vi "TLB Native Dynamic Events ver 0.26e.vi"() -> ()   [LabVIEW 2018] (continued)
      tunnel: [w3002 w3015 w3027 w3042 w3061 w3076 w3091 w3105 w3119 w3135 w3150 w3164 w3175 w3192 w3210 w3228 w3251 w3263 w3276 w3305 w3318 w3331 w3346 w3357 w3373 w3393 w3428 w3462 w3475 w3488 w3499 w3511 w3527 w3543 w3555 w3568 w3602 w3613 w3625 w3657 w3668 w3679 w3692 w3705 w3718 w3731 w3744 w3759 w3775 w3788 w3804 w3820 w3836 w3853 w3866 w3886 w3906] -> w237
      tunnel: [_ _ _ _ _ _ _ _ _ _ _ _ _ _ _ _ _ _ _ _ _ _ _ _ _ _ _ _ _ _ _ _ _ _ _ w3567 w3597 _ _ _ _ _ _ _ _ _ _ _ _ _ _ _ _ _ _ _ _] -> w235
      tunnel: w233 -> [w3001 w3014 w3026 w3041 w3060 w3075 w3090 w3104 w3118 w3134 w3149 w3163 w3174 w3191 w3209 w3227 w3243 w3262 w3274 w3304 w3317 w3330 w3345 w3356 w3375 w3395 w3430 w3461 w3474 w3487 w3498 w3510 w3526 w3542 w3554 w3566 w3601 w3612 w3624 w3656 w3667 w3678 w3691 w3704 w3717 w3730 w3743 w3758 w3774 w3787 w3803 w3819 w3835 w3852 w3865 w3885 w3905]
      tunnel: [w3001 w3014 w3026 w3041 w3060 w3075 w3090 w3104 w3118 w3134 w3149 w3163 w3174 w3191 w3209 w3227 w3243 w3262 w3274 w3304 w3317 w3330 w3345 w3356 w3375 w3395 w3430 w3461 w3474 w3487 w3498 w3510 w3526 w3542 w3554 w3566 w3601 w3612 w3624 w3656 w3667 w3678 w3691 w3704 w3717 w3730 w3743 w3758 w3774 w3787 w3803 w3819 w3835 w3852 w3865 w3885 w3905] -> w232
      tunnel: w228 -> [w3000 w3013 w3025 w3040 w3059 w3074 w3089 w3103 w3117 w3133 w3148 w3162 w3173 w3190 w3208 w3224 w3242 w3261 w3273 w3303 w3316 w3329 w3344 w3355 w3370 w3388 w3423 w3460 w3473 w3486 w3497 w3509 w3525 w3541 w3553 w3565 w3595 w3611 w3623 w3655 w3666 w3677 w3690 w3703 w3716 w3729 w3742 w3757 w3773 w3786 w3802 w3818 w3834 w3851 w3864 w3884 w3899]
      tunnel: [w3000 w3013 w3025 w3040 w3059 w3074 w3089 w3103 w3117 w3133 w3148 w3162 w3173 w3190 w3208 w3224 w3242 w3261 w3273 w3303 w3316 w3329 w3344 w3355 w3369 w3388 w3423 w3460 w3473 w3486 w3497 w3509 w3525 w3541 w3553 w3565 w3588 w3611 w3623 w3654 w3666 w3677 w3690 w3703 w3716 w3729 w3742 w3757 w3773 w3786 w3802 w3818 w3834 w3851 w3864 w3884 w3898] -> w227
      frame "Exit" {
        # ">>State Logic  >>"
        # ">>> Time cluster >>>"
        # ">>> Yaw >>>"
        # ">>> Stepper position >>>"
        # ">>> Encoders >>>"
        # ">>> Object detection >>>"
        # ">>> Ultrasonic Sensors Detect >>>"
        n75 = call "Imaq Dispose"("All Images? (No)"=TRUE) -> ()  [unwired: 5 in, 1 out]
      }
      frame "----Movement States----" {
        # ">>State Logic  >>"
        # ">>> Time cluster >>>"
        # ">>> Yaw >>>"
        # ">>> Stepper position >>>"
        # ">>> Encoders >>>"
        # ">>> Object detection >>>"
        # ">>> Ultrasonic Sensors Detect >>>"
      }
      frame "FORWARD" {
        # ">>State Logic  >>"
        # ">>> Time cluster >>>"
        # ">>> Yaw >>>"
        # ">>> Stepper position >>>"
        # ">>> Encoders >>>"
        # ">>> Object detection >>>"
        # ">>> Ultrasonic Sensors Detect >>>"
        n76 = Unbundle By Name(w3033) -> ("Yaw"=w3029:dbl)
        n77 = call "MOTOR CONTROL WITH PID AE.vi"("Yaw"=w3029, "Speed"=40.0, "Direction"=MOTOR_CONTROL_WITH_PID_AE_DIRECTION_TYPE_DEF."y-axis movement", "AE Mode"=MOTOR_CONTROL_WITH_PID_AE_DATA_MODE_TYPE_DEF."Write to AE") -> ()  [unwired: 1 out]
      }
      frame "FORWARD - IR ASSIST" {
        # "Algorithm sensitivity"
        # "Distance to maintain from wall"
        # ">>State Logic  >>"
        # ">>> Time cluster >>>"
        # ">>> Yaw >>>"
        # ">>> Stepper position >>>"
        # ">>> Encoders >>>"
        # ">>> Object detection >>>"
        # ">>> Ultrasonic Sensors Detect >>>"
        n78 = Unbundle By Name(w3048) -> ("Left IR Sensor"=w3047:dbl)
        n79 = Subtract(x=w3047, y=10.0) -> (x-y=w3045:dbl)
        n80 = Multiply(x=w3045, y=0.2) -> (x*y=w3043:dbl)
        n81 = call "MOTOR CONTROL WITH PID AE.vi"("Yaw"=w3043, "Speed"=35.0, "Direction"=MOTOR_CONTROL_WITH_PID_AE_DIRECTION_TYPE_DEF."y-axis movement", "AE Mode"=MOTOR_CONTROL_WITH_PID_AE_DATA_MODE_TYPE_DEF."Write to AE") -> ()  [unwired: 1 out]
      }
      frame "LEFT" {
        # ">>State Logic  >>"
        # ">>> Time cluster >>>"
        # ">>> Yaw >>>"
        # ">>> Stepper position >>>"
        # ">>> Encoders >>>"
        # ">>> Object detection >>>"
        # ">>> Ultrasonic Sensors Detect >>>"
        n82 = Unbundle By Name(w3067) -> ("Yaw"=w3064:dbl)
        n83 = call "MOTOR CONTROL WITH PID AE.vi"("Yaw"=w3064, "Speed"=-20.0, "Direction"=MOTOR_CONTROL_WITH_PID_AE_DIRECTION_TYPE_DEF."x-axis movement", "AE Mode"=MOTOR_CONTROL_WITH_PID_AE_DATA_MODE_TYPE_DEF."Write to AE") -> ()  [unwired: 1 out]
      }
      frame "RIGHT" {
        # ">>> Time cluster >>>"
        # ">>> Yaw >>>"
        # ">>> Stepper position >>>"
        # ">>> Encoders >>>"
        # ">>> Object detection >>>"
        # ">>> Ultrasonic Sensors Detect >>>"
        n84 = Unbundle By Name(w3082) -> ("Yaw"=w3078:dbl)
        n85 = call "MOTOR CONTROL WITH PID AE.vi"("Yaw"=w3078, "Speed"=30.0, "Direction"=MOTOR_CONTROL_WITH_PID_AE_DIRECTION_TYPE_DEF."x-axis movement", "AE Mode"=MOTOR_CONTROL_WITH_PID_AE_DATA_MODE_TYPE_DEF."Write to AE") -> ()  [unwired: 1 out]
      }
      frame "R-ACW" {
        # ">>> IR Sensors >>>"
        # ">>> Time cluster >>>"
        # ">>> Yaw >>>"
        # ">>> Stepper position >>>"
        # ">>> Encoders >>>"
        # ">>> Object detection >>>"
        # ">>> Ultrasonic Sensors Detect >>>"
        n86 = call "MOTOR CONTROL WITH PID AE.vi"("Speed"=10.0, "Direction"=MOTOR_CONTROL_WITH_PID_AE_DIRECTION_TYPE_DEF."rotation", "AE Mode"=MOTOR_CONTROL_WITH_PID_AE_DATA_MODE_TYPE_DEF."Write to AE") -> ()  [unwired: 1 in, 1 out]
      }
      frame "R-CW" {
        (unwired) -0.2 ("Speed")
        # ">>> Time cluster >>>"
        # ">>> Yaw >>>"
        # ">>> Stepper position >>>"
        # ">>> Encoders >>>"
        # ">>> Object detection >>>"
        # ">>> Ultrasonic Sensors Detect >>>"
        n87 = call "MOTOR CONTROL WITH PID AE.vi"("Speed"=-10.0, "Direction"=MOTOR_CONTROL_WITH_PID_AE_DIRECTION_TYPE_DEF."rotation", "AE Mode"=MOTOR_CONTROL_WITH_PID_AE_DATA_MODE_TYPE_DEF."Write to AE") -> ()  [unwired: 1 in, 1 out]
      }
      frame "X AXIS - SLOW" {
        # ">>> Line Sensor Cluster>>>"
        # ">>> IR Sensors >>>"
        # ">>> Time cluster >>>"
        # ">>> Yaw >>>"
        # ">>> Stepper position >>>"
        # ">>> Encoders >>>"
        # ">>> Object detection >>>"
        # ">>> Ultrasonic Sensors Detect >>>"
        n88 = Unbundle By Name(w3121) -> ("xSpeed"=w3120:dbl)
        n89 = Unbundle By Name(w3126) -> ("Yaw"=w3123:dbl)
        n90 = call "MOTOR CONTROL WITH PID AE.vi"("Yaw"=w3123, "Speed"=w3120, "Direction"=MOTOR_CONTROL_WITH_PID_AE_DIRECTION_TYPE_DEF."x-axis movement", "AE Mode"=MOTOR_CONTROL_WITH_PID_AE_DATA_MODE_TYPE_DEF."Write to AE") -> ()  [unwired: 1 out]
      }
      frame "REVERSE" {
        # ">>> Time cluster >>>"
        # ">>> Yaw >>>"
        # ">>> Stepper position >>>"
        # ">>> Encoders >>>"
        # ">>> Object detection >>>"
        # ">>> Ultrasonic Sensors Detect >>>"
        n91 = Unbundle By Name(w3141) -> ("Yaw"=w3137:dbl)
        n92 = call "MOTOR CONTROL WITH PID AE.vi"("Yaw"=w3137, "Speed"=-50.0, "Direction"=MOTOR_CONTROL_WITH_PID_AE_DIRECTION_TYPE_DEF."y-axis movement", "AE Mode"=MOTOR_CONTROL_WITH_PID_AE_DATA_MODE_TYPE_DEF."Write to AE") -> ()  [unwired: 1 out]
      }
      frame "STOP" {
        n93 = Wait (ms)(milliseconds to wait=u32 100) -> ()  [unwired: 1 out]
        n94 = call "MOTOR CONTROL WITH PID AE.vi"("Direction"=MOTOR_CONTROL_WITH_PID_AE_DIRECTION_TYPE_DEF."stop", "AE Mode"=MOTOR_CONTROL_WITH_PID_AE_DATA_MODE_TYPE_DEF."Write to AE") -> ()  [unwired: 2 in, 1 out]
      }
      frame "----SENSOR READING---- " {
      }
      frame "READ ENCODERS" {
        # ">>> Time cluster >>>"
        # ">>> Yaw >>>"
        # ">>> Stepper position >>>"
        # ">>> Object detection >>>"
        # ">>> Current encoder distance >>>"
        # ">>> Ultrasonic Sensors Detect >>>"
        n95 = call "MOTOR CONTROL WITH PID AE.vi"("AE Mode"=MOTOR_CONTROL_WITH_PID_AE_DATA_MODE_TYPE_DEF."Read from AE") -> ("Speed & distance"=w3180:T15)  [unwired: 3 in]
        n96 = Unbundle By Name(w3180) -> ("xDistance"=w3179:dbl, "yDistance"=w3178:dbl, "wDistance"=w3177:dbl)
        n97 = Bundle By Name(cluster=w3187, "xDistance"=w3179, "yDistance"=w3178, "wDistance"=w3177) -> (w3186:T8)
      }
      frame "READ ULTRASONIC" {
        (unwired) navX_type_def."Read Values" ("Mode")
        (unwired) MOTOR_CONTROL_NO_PID_Type_Def."Latch" ("Direction")
        # ">>> Line Sensor Cluster>>>"
        # ">>> IR Sensors >>>"
        # ">>State Logic  >>"
        # ">>> Time cluster >>>"
        # ">>> Ultrasonic Sensors Detect >>>"
        # ">>> Object detection >>>"
        # ">>> Encoders >>>"
        # ">>> Stepper position >>>"
        # ">>> Yaw >>>"
        n98 = call "Arduino Interfacing VI.vi"("AE Mode"=Arduino_Interfacing."Read From Arduino") -> ("Arduino Data"=w3200:T17)  [unwired: 3 in, 1 out]
        n99 = Unbundle By Name(w3200) -> ("PING A"=w3199:u8, "PING B"=w3198:u8, "PING C"=w3197:u8, "PING D"=w3196:u8)
        n100 = Bundle By Name(cluster=w3206, "PING_A"=w3199, "PING_B"=w3198, "PING_C"=w3197, "PING_D"=w3196) -> (w3207:T9)
      }
      frame "READ NAVX" {
        # ">> Item Selection Bias >>"
        # ">>State Logic  >>"
        # ">>> Line Sensor Cluster>>>"
        # ">>> IR Sensors >>>"
        # ">>> Time cluster >>>"
        # ">>> Yaw >>>"
        # ">>> Ultrasonic Sensors Detect >>>"
        # ">>> Object detection >>>"
        # ">>> Encoders >>>"
        # ">>> Stepper position >>>"
        n101 = call "navX reading VI.vi"("Mode"=navX_type_def."Read Values") -> ("NavX Readings"=w3213:T16)  [unwired: 2 in, 3 out]
        n102 = Unbundle By Name(w3213) -> ("Heading"=w3212:dbl)
        n103 = Unbundle By Name(w3213) -> ("Yaw"=w3216:dbl)
        n104 = Bundle By Name(cluster=w3218, "Yaw"=w3216, "Compass"=w3212) -> (w3217:T6)
      }
      frame "READ IR" {
        w3226 = T41 [enum."B/AI2"] items=["Not Connected", "AudioIn/Left", "AudioIn/Right", "C/AI0", "C/AI1", "A/AI0", "A/AI1", "A/AI2", "A/AI3", "A/AI4", "A/AI5", "A/AI6", "A/AI7", "B/AI0", "B/AI1", "B/AI2", "B/AI3", "B/AI4", "B/AI5", "B/AI6", "B/AI7", "AI/AI0", "AI/AI1", "AI/AI2", "AI/AI3", "A/AI0 (DIFF)", "A/AI1 (DIFF)", "A/AI2 (DIFF)", "A/AI3 (DIFF)", "B/AI0 (DIFF)", "B/AI1 (DIFF)", "B/AI2 (DIFF)", "B/AI3 (DIFF)"] ("AI Channel")
        w3230 = T41 [enum."B/AI1"] items=["Not Connected", "AudioIn/Left", "AudioIn/Right", "C/AI0", "C/AI1", "A/AI0", "A/AI1", "A/AI2", "A/AI3", "A/AI4", "A/AI5", "A/AI6", "A/AI7", "B/AI0", "B/AI1", "B/AI2", "B/AI3", "B/AI4", "B/AI5", "B/AI6", "B/AI7", "AI/AI0", "AI/AI1", "AI/AI2", "AI/AI3", "A/AI0 (DIFF)", "A/AI1 (DIFF)", "A/AI2 (DIFF)", "A/AI3 (DIFF)", "B/AI0 (DIFF)", "B/AI1 (DIFF)", "B/AI2 (DIFF)", "B/AI3 (DIFF)"] ("AI Channel")
        w3235 = T41 [enum."B/AI0"] items=["Not Connected", "AudioIn/Left", "AudioIn/Right", "C/AI0", "C/AI1", "A/AI0", "A/AI1", "A/AI2", "A/AI3", "A/AI4", "A/AI5", "A/AI6", "A/AI7", "B/AI0", "B/AI1", "B/AI2", "B/AI3", "B/AI4", "B/AI5", "B/AI6", "B/AI7", "AI/AI0", "AI/AI1", "AI/AI2", "AI/AI3", "A/AI0 (DIFF)", "A/AI1 (DIFF)", "A/AI2 (DIFF)", "A/AI3 (DIFF)", "B/AI0 (DIFF)", "B/AI1 (DIFF)", "B/AI2 (DIFF)", "B/AI3 (DIFF)"] ("AI Channel")
        # ">>> Line Sensor Cluster>>>"
        # ">>> IR Sensors >>>"
        # ">>State Logic  >>"
        # ">>> Time cluster >>>"
        # ">>> Ultrasonic Sensors Detect >>>"
        # ">>> Object detection >>>"
        # ">>> Encoders >>>"
        # ">>> Stepper position >>>"
        # ">>> Yaw >>>"
        n105 = call <vilib>:"Sharp IR.vi"("AI Channel"=w3235) -> ("Sharp IR Distance"=w3231:dbl)  [unwired: 8 in, 2 out]
        n106 = call <vilib>:"Sharp IR.vi"("AI Channel"=w3230) -> ("Sharp IR Distance"=w3229:dbl)  [unwired: 8 in, 2 out]
        n107 = call <vilib>:"Sharp IR.vi"("AI Channel"=w3226) -> ("Sharp IR Distance"=w3225:dbl)  [unwired: 8 in, 2 out]
        n108 = Bundle By Name(cluster=w3233, "Left IR Sensor"=w3231, "Arm IR Sensor"=w3229, "Bottom IR Sensor"=w3225) -> (w3232:T5)
      }
      frame "READ LINE SENSOR" {
        # ">>> IR Sensors >>>"
        # ">>> Line Sensor Cluster>>>"
        # ">>State Logic  >>"
        # ">>> Time cluster >>>"
        # ">>> Object detection >>>"
        # ">>> Yaw >>>"
        # ">>> Ultrasonic Sensors Detect >>>"
        # ">>> Encoders >>>"
        # ">>> Stepper position >>>"
        n109 = call "Line Sensor AE.vi"("AE State"=Line_Sensor_AE_Type_Def."READ FROM LINE SENSORS") -> ("Line Detected?"=w3249:bool, "Line Sensor Raw Values"=w3248:T43)
        n110 = Unbundle By Name(w3248) -> ("S1"=w3247:dbl, "S2"=w3246:dbl, "S3"=w3245:dbl, "S4"=w3244:dbl)
        n111 = Bundle By Name(cluster=w3252, "Line Detected?"=w3249, "S1"=w3247, "S2"=w3246, "S3"=w3245, "S4"=w3244) -> (w3251:T4)
      }
      frame "----SYSTEM MODES----" {
        (unwired) I2C_MASTER_Type_Def."Last State" ("Arduino Mode")
        # ">>> Object detection >>>"
        # ">>> Yaw >>>"
        # ">>> Ultrasonic Sensors Detect >>>"
        # ">>> Encoders >>>"
        # ">>> Stepper position >>>"
      }
      frame "INIT" {
        w3296 = u8 0
        w3297 = 0.0
        # ">>> IR Sensors >>>"
        # ">>> IR Sensors >>>"
        # ">>> Line Sensor Cluster>>>"
        # ">>> Time cluster >>>"
        # ">>> Object detection >>>"
        # ">>> Yaw >>>"
        # ">>> Ultrasonic Sensors Detect >>>"
        # ">>> Encoders >>>"
        # ">>> Stepper position >>>"
        # ">>State Logic  >>"
        n112 = call "Arduino Interfacing VI.vi"("AE Mode"=Arduino_Interfacing."Initialize") -> ()  [unwired: 3 in, 2 out]
        n113 = call "FGV Stop.vi"("Init/Read/Write State"=States_for_Action_Engine."Initialize") -> ()  [unwired: 2 in, 2 out]
        n114 = call "Elasped Timer.vi"("Action"=Elapsed_timer_control."Initialize") -> ()  [unwired: 7 in, 4 out]
        n115 = call "MOTOR CONTROL WITH PID AE.vi"("AE Mode"=MOTOR_CONTROL_WITH_PID_AE_DATA_MODE_TYPE_DEF."Init AE") -> ()  [unwired: 3 in, 1 out]
        n116 = call "IMAQ Reference AE.vi"("IMAQ AE States"=IMAQ_Reference_AE."Initialize AE") -> ()  [unwired: 1 in, 2 out]
        n117 = call "Line Sensor AE.vi"("AE State"=Line_Sensor_AE_Type_Def."INIT AE") -> ()  [unwired: 2 out]
        n118 = Bundle By Name(cluster=w3290, "Recognized Object"=FALSE, "Object X coordinate"=0.0, "Object Y coordinate"=0.0) -> (w3289:T11)
        n119 = Bundle By Name(cluster=w3295, "y Stepper Position"=u8 0, "z Stepper Position"=u8 0) -> (w3294:T7)
        n120 = Bundle By Name(cluster=w3299, "xDistance"=w3297, "yDistance"=w3297, "wDistance"=w3297) -> (w3298:T8)
        n121 = Bundle By Name(cluster=w3301, "PING_A"=w3296, "PING_B"=w3296, "PING_C"=w3296, "PING_D"=w3296) -> (w3302:T9)
        n122 = invoke class="VI" method="Default Vals.Reinit All"() -> ()  [unwired: 3 in, 3 out]
        n123 = Bundle By Name(cluster=w3285, "Yaw"=0.0) -> (w3284:T6)
        n124 = call "Box Colour FGV.vi"("Init/R/W State"=Box_Colour_FGV_States."Initialize") -> ()  [unwired: 9 in, 2 out]
      }
      frame "ARDUINO - ULTRASONIC" {
        # ">>> Time cluster >>>"
        # ">>> Line Sensor Cluster>>>"
        # ">>> Object detection >>>"
        # ">>> Yaw >>>"
        # ">>> Ultrasonic Sensors Detect >>>"
        # ">>> Encoders >>>"
        # ">>> Stepper position >>>"
        # ">>State Logic  >>"
        n125 = call "Arduino Interfacing VI.vi"("Data to Write"=I2C_MASTER_WRITE_NEW_Type_Def."Ultrasonic sensors", "AE Mode"=Arduino_Interfacing."Write to Arduino") -> ()  [unwired: 2 in, 2 out]
      }
      frame "NAVX CALIBRATE" {
        # ">>> Object detection >>>"
        # ">>> Yaw >>>"
        # ">>> Ultrasonic Sensors Detect >>>"
        # ">>> Encoders >>>"
        # ">>> Stepper position >>>"
        # ">>State Logic  >>"
        # "Adds a 15 second delay to the startup process \nfor the NavX to calibrate"
        n126 = Wait (ms)(milliseconds to wait=u32 1000) -> ()  [unwired: 1 out]
      }
      frame "NO ACTION", Default {
        (unwired) u8 0 ("y Stepper value")
        (unwired) TRUE ("Latch")
        (unwired) navX_type_def."Read Values" ("Mode")
        (unwired) MOTOR_CONTROL_NO_PID_Type_Def."Latch" ("Direction")
        # ">>> Object detection >>>"
        # ">>> Yaw >>>"
        # ">>> Ultrasonic Sensors Detect >>>"
        # ">>> Encoders >>>"
        # ">>> Stepper position >>>"
        # ">>State Logic  >>"
        n127 = case shown="4" w3338 {
          tunnel: [0 100] -> w3340
          frame 1, Default {
          }
          frame 4 {
          }
        }
      }
      frame "----RESET CASES----" {
        (unwired) I2C_MASTER_Type_Def."Last State" ("Arduino Mode")
        # ">>> Object detection >>>"
        # ">>> Yaw >>>"
        # ">>> Ultrasonic Sensors Detect >>>"
        # ">>> Encoders >>>"
        # ">>> Stepper position >>>"
        # ">>State Logic  >>"
      }
      frame "RESET ENCODERS" {
        # ">>> Object detection >>>"
        # ">>> Yaw >>>"
        # ">>> Ultrasonic Sensors Detect >>>"
        # ">>> Encoders >>>"
        # ">>> Stepper position >>>"
        # ">>State Logic  >>"
        n128 = call "MOTOR CONTROL WITH PID AE.vi"("Direction"=MOTOR_CONTROL_WITH_PID_AE_DIRECTION_TYPE_DEF."reset encoders", "AE Mode"=MOTOR_CONTROL_WITH_PID_AE_DATA_MODE_TYPE_DEF."Write to AE") -> ()  [unwired: 2 in, 1 out]
      }
      frame "RESET FLAGS" {
        w3368 = FALSE ("Line Detected?")
        # ">>> Line Sensor Cluster>>>"
        # ">>> IR Sensors >>>"
        # ">>> Time cluster >>>"
        # ">>> Object detection >>>"
        # ">>> Yaw >>>"
        # ">>> Ultrasonic Sensors Detect >>>"
        # ">>> Encoders >>>"
        # ">>> Stepper position >>>"
        # ">>> Line Sensor Cluster>>>"
        # ">>> IR Sensors >>>"
        # ">>> Time cluster >>>"
        # ">>> Object detection >>>"
        # ">>> Yaw >>>"
        # ">>> Ultrasonic Sensors Detect >>>"
        # ">>> Encoders >>>"
        # ">>> Stepper position >>>"
        # "Resets BOOLEAN FLAGS only"
        n129 = Wait (ms)(milliseconds to wait=u32 20) -> ()  [unwired: 1 out]
        n130 = Bundle By Name(cluster=w3384, "Recognized Object"=FALSE) -> (w3383:T11)
        n131 = Bundle By Name(cluster=w3374, "Line Detected?"=FALSE) -> (w3373:T4)
        n132 = Bundle By Name(cluster=w3378, "Time up flag"=FALSE) -> (w3377:T3)
        n133 = Bundle By Name(cluster=w3370, "Red"=w3368, "Black"=w3368, "Blue"=w3368, "Yellow"=w3368, "Green"=w3368, "Unknown"=w3368, "Image processing done"=w3368) -> (w3369:T1)
      }
      frame "RESET SENSOR VALUES" {
        w3389 = 0.0 ("S4")
        w3390 = 0.0 ("S4")
        # "Resets SENSOR VALUES only"
        # ">>> Line Sensor Cluster>>>"
        # ">>> IR Sensors >>>"
        # ">>> Time cluster >>>"
        # ">>> Object detection >>>"
        # ">>> Yaw >>>"
        # ">>> Ultrasonic Sensors Detect >>>"
        # ">>> Encoders >>>"
        # ">>> Stepper position >>>"
        # ">>> Line Sensor Cluster>>>"
        # ">>> IR Sensors >>>"
        # ">>> Time cluster >>>"
        # ">>> Object detection >>>"
        # ">>> Yaw >>>"
        # ">>> Ultrasonic Sensors Detect >>>"
        # ">>> Encoders >>>"
        # ">>> Stepper position >>>"
        # "Resets any software variables\nand/or non-critical states"
        n134 = Wait (ms)(milliseconds to wait=u32 20) -> ()  [unwired: 1 out]
        n135 = Bundle By Name(cluster=w3398, "SET TIME TO CHECK"=0.0) -> (w3397:T3)
        n136 = Bundle By Name(cluster=w3414, "Object X coordinate"=0.0, "Object Y coordinate"=0.0) -> (w3413:T11)
        n137 = Bundle By Name(cluster=w3405, "y Stepper Position"=u8 0, "z Stepper Position"=u8 0) -> (w3404:T7)
        n138 = Bundle By Name(cluster=w3392, "Left IR Sensor"=w3389, "Arm IR Sensor"=w3389) -> (w3391:T5)
        n139 = Bundle By Name(cluster=w3410, "xDistance"=0.0, "yDistance"=0.0, "wDistance"=0.0) -> (w3409:T8)
        n140 = Bundle By Name(cluster=w3421, "PING_A"=u8 0, "PING_B"=u8 0, "PING_C"=u8 0, "PING_D"=u8 0) -> (w3420:T9)
        n141 = Bundle By Name(cluster=w3401, "Yaw"=0.0) -> (w3400:T6)
        n142 = Bundle By Name(cluster=w3394, "S1"=w3390, "S2"=w3390, "S3"=w3390, "S4"=w3390) -> (w3393:T4)
      }
      frame "RESET ALL SENSORS" {
        w3424 = 0.0 ("SET TIME TO CHECK")
        # ">>> Line Sensor Cluster>>>"
        # ">>> IR Sensors >>>"
        # ">>> Time cluster >>>"
        # ">>> Object detection >>>"
        # ">>> Yaw >>>"
        # ">>> Ultrasonic Sensors Detect >>>"
        # ">>> Encoders >>>"
        # ">>> Stepper position >>>"
        # ">>> Line Sensor Cluster>>>"
        # ">>> IR Sensors >>>"
        # ">>> Time cluster >>>"
        # ">>> Object detection >>>"
        # ">>> Yaw >>>"
        # ">>> Ultrasonic Sensors Detect >>>"
        # ">>> Encoders >>>"
        # ">>> Stepper position >>>"
        # "Resets ALL SENSOR PARAMTERS"
        n143 = Wait (ms)(milliseconds to wait=u32 20) -> ()  [unwired: 1 out]
        n144 = Bundle By Name(cluster=w3434, "Time up flag"=FALSE, "SET TIME TO CHECK"=0.0) -> (w3433:T3)
        n145 = Bundle By Name(cluster=w3451, "Recognized Object"=FALSE, "Object X coordinate"=0.0, "Object Y coordinate"=0.0) -> (w3450:T11)
        n146 = Bundle By Name(cluster=w3441, "y Stepper Position"=u8 0, "z Stepper Position"=u8 0) -> (w3440:T7)
        n147 = Bundle By Name(cluster=w3429, "Line Detected?"=FALSE) -> (w3428:T4)
        n148 = Bundle By Name(cluster=w3426, "Left IR Sensor"=w3424, "Arm IR Sensor"=w3424) -> (w3425:T5)
        n149 = Bundle By Name(cluster=w3446, "xDistance"=0.0, "yDistance"=0.0, "wDistance"=0.0) -> (w3445:T8)
        n150 = Bundle By Name(cluster=w3458, "PING_A"=u8 0, "PING_B"=u8 0, "PING_C"=u8 0, "PING_D"=u8 0) -> (w3457:T9)
        n151 = Bundle By Name(cluster=w3437, "Yaw"=0.0) -> (w3436:T6)
      }
      frame "RESET YAW" {
        n152 = Wait (ms)(milliseconds to wait=u32 100) -> ()  [unwired: 1 out]
        n153 = call "navX reading VI.vi"("Mode"=navX_type_def."Zero Yaw") -> ()  [unwired: 2 in, 4 out]
      }
      frame "RESET ARM" {
        n154 = call "Arduino Interfacing VI.vi"("Data to Write"=I2C_MASTER_WRITE_NEW_Type_Def."Soft Reset", "AE Mode"=Arduino_Interfacing."Write to Arduino") -> ()  [unwired: 2 in, 2 out]
      }
      frame "--------CAM STATES-------" {
      }
      frame "OPEN IMAQ REF" {
        # ">>> Line Sensor Cluster>>>"
        # ">>State Logic  >>"
        # ">>> Time cluster >>>"
        # ">>> Object detection >>>"
        # ">>> Yaw >>>"
        # ">>> Ultrasonic Sensors Detect >>>"
        # ">>> Encoders >>>"
        # ">>> Stepper position >>>"
        # ">>> IR Sensors >>>"
        n155 = call "IMAQ Reference AE.vi"("IMAQ AE States"=IMAQ_Reference_AE."Initialize AE") -> ()  [unwired: 1 in, 2 out]
      }
      frame "OPEN LOG CAM" {
        n156 = call "Webcam AE.vi"("Session In"=T39 "cam0", "Camera states"=Webcam_AE."Initialize Camera") -> ("error out"=w3515:errorcluster, "Session Out"=w3514:T39)  [unwired: 1 in, 1 out]
        n157 = call "Webcam AE.vi"("error in (no error)"=w3515, "Session In"=w3514, "Camera states"=Webcam_AE."Open Camera") -> ()  [unwired: 3 out]
      }
      frame "OPEN LIFE CAM" {
        n158 = call "Webcam AE.vi"("Session In"=T39 "cam1", "Camera states"=Webcam_AE."Initialize Camera") -> ("error out"=w3531:errorcluster, "Session Out"=w3530:T39)  [unwired: 1 in, 1 out]
        n159 = call "Webcam AE.vi"("error in (no error)"=w3531, "Session In"=w3530, "Camera states"=Webcam_AE."Open Camera") -> ()  [unwired: 3 out]
      }
      frame "CAM ACQ" {
        # ">>State Logic  >>"
        # ">>> Time cluster >>>"
        # ">>> Yaw >>>"
        # ">>> Stepper position >>>"
        # ">>> Encoders >>>"
        # ">>> Object detection >>>"
        # ">>> Ultrasonic Sensors Detect >>>"
        n160 = call "Webcam AE.vi"("Camera states"=Webcam_AE."Continuous Acquisition") -> ()  [unwired: 2 in, 3 out]
      }
      frame "CAM CLOSE" {
        # ">>> Box Colour Detection >>>"
        # ">>> Line Sensor Cluster>>>"
        # ">>> IR Sensors >>>"
        # ">>State Logic  >>"
        # ">>> Time cluster >>>"
        # ">>> Yaw >>>"
        # ">>> Stepper position >>>"
        # ">>> Encoders >>>"
        # ">>> Object detection >>>"
        # ">>> Ultrasonic Sensors Detect >>>"
        n161 = call "Webcam AE.vi"("Camera states"=Webcam_AE."Close Camera") -> ()  [unwired: 2 in, 3 out]
      }
      frame "PROCESS IMAGE" {
        # ">>> Line Sensor Cluster>>>"
        # ">>> IR Sensors >>>"
        # ">> Item Selection Bias >>"
        # ">> Item Selection Bias >>"
        # ">>State Logic  >>"
        # ">>> Time cluster >>>"
        # ">>> Yaw >>>"
        # ">>> Stepper position >>>"
        # ">>> Encoders >>>"
        # ">>> Object detection >>>"
        # ">>> Ultrasonic Sensors Detect >>>"
        n162 = call "Webcam AE.vi"("Camera states"=Webcam_AE."Retrieve Image") -> ("error out"=w3579:errorcluster, "Image Out"=w3580:T45)  [unwired: 2 in, 1 out]
        n163 = call "IMAQ Reference AE.vi"("IMAQ AE States"=IMAQ_Reference_AE."Get IMAQ Reference") -> ("Image Out"=w3569:T45)  [unwired: 1 in, 1 out]
        n164 = call "Object Detection SubVI.vi"("Error In"=w3579, "Mode"=w3566, "Image Dest"=w3569, "Image in"=w3580) -> ("Error out"=w3567:errorcluster, "Object Center Coordinates"=w3576:cluster{"x":sgl, "y":sgl}, "Object detection cluster"=w3572:T46)  [unwired: 1 out]
        n165 = Unbundle By Name(w3572) -> ("Object detected?"=w3573:bool)
        n166 = Unbundle By Name(w3576) -> ("x"=w3575:sgl, "y"=w3574:sgl)
        n167 = Bundle By Name(cluster=w3578, "Recognized Object"=w3573, "Object X coordinate"=w3575, "Object Y coordinate"=w3574) -> (w3577:T11)
      }
      frame "COLOUR PROCESSING" {
        # ">>> Box Colour Detection >>>"
        # ">>> Box Colour Detection >>>"
        # ">>> Line Sensor Cluster>>>"
        # ">>> IR Sensors >>>"
        # ">> Item Selection Bias >>"
        # ">> Item Selection Bias >>"
        # ">>State Logic  >>"
        # ">>> Time cluster >>>"
        # ">>> Yaw >>>"
        # ">>> Stepper position >>>"
        # ">>> Encoders >>>"
        # ">>> Object detection >>>"
        # ">>> Ultrasonic Sensors Detect >>>"
        n168 = call "Webcam AE.vi"("Camera states"=Webcam_AE."Retrieve Image") -> ("error out"=w3598:errorcluster, "Image Out"=w3599:T45)  [unwired: 2 in, 1 out]
        n169 = call "Box Colour Detection SubVI.vi"("Image In"=w3599, "Error In"=w3598) -> ("Colour output boolean cluster"=w3596:T47, "Error out"=w3597:errorcluster)  [unwired: 1 out]
        n170 = Unbundle By Name(w3596) -> ("Red"=w3594:bool, "Black"=w3593:bool, "Blue"=w3592:bool, "Yellow"=w3591:bool, "Green"=w3590:bool, "No recognizable coolour"=w3589:bool)
        n171 = Bundle By Name(cluster=w3595, "Red"=w3594, "Black"=w3593, "Blue"=w3592, "Yellow"=w3591, "Green"=w3590, "Unknown"=w3589) -> (w3588:T1)
      }
      frame "DISPOSE CAM BUFFERS" {
        # ">> Item Selection Bias >>"
        # ">>> Line Sensor Cluster>>>"
        # ">>> IR Sensors >>>"
        # ">>State Logic  >>"
        # ">>> Time cluster >>>"
        # ">>> Yaw >>>"
        # ">>> Stepper position >>>"
        # ">>> Encoders >>>"
        # ">>> Object detection >>>"
        # ">>> Ultrasonic Sensors Detect >>>"
        n172 = call "Webcam AE.vi"("Camera states"=Webcam_AE."Dispose Camera Image Buffer") -> ()  [unwired: 2 in, 3 out]
      }
      frame "DISPOSE PROC BUFFERS" {
        # ">>> Box Colour Detection >>>"
        # ">>> Line Sensor Cluster>>>"
        # ">>State Logic  >>"
        # ">>> IR Sensors >>>"
        # ">>> Time cluster >>>"
        # ">>> Object detection >>>"
        # ">>> Yaw >>>"
        # ">>> Ultrasonic Sensors Detect >>>"
        # ">>> Encoders >>>"
        # ">>> Stepper position >>>"
        n173 = call "IMAQ Reference AE.vi"("IMAQ AE States"=IMAQ_Reference_AE."Dispose Processing Buffer") -> ()  [unwired: 1 in, 2 out]
      }
      frame "BOX COLOUR" {
        # ">>> Box Colour Detection >>>"
        # ">>> Line Sensor Cluster>>>"
        # ">>State Logic  >>"
        # ">>> IR Sensors >>>"
        # ">>> Time cluster >>>"
        # ">>> Object detection >>>"
        # ">>> Yaw >>>"
        # ">>> Ultrasonic Sensors Detect >>>"
        # ">>> Encoders >>>"
        # ">>> Stepper position >>>"
        n174 = call "Box Colour Detection Sequence.vi"() -> ("Colour scan time out?"=w3651:bool, "Colour output boolean cluster"=w3653:T47)  [unwired: 9 in, 1 out]
        n175 = Unbundle By Name(w3653) -> ("Red"=w3650:bool, "Black"=w3646:bool, "Blue"=w3643:bool, "Yellow"=w3642:bool, "Green"=w3639:bool, "No recognizable coolour"=w3652:bool)
        n176 = Select(t=Box_Colour_FGV_Colours."Green" ("Colour"), s=w3639, f=Box_Colour_FGV_Colours."None" ("Colour")) -> (s? t:f=w3637:T2)
        n177 = Select(t=Box_Colour_FGV_Colours."Yellow" ("Colour"), s=w3642, f=w3637) -> (s? t:f=w3636:T2)
        n178 = Select(t=Box_Colour_FGV_Colours."Blue" ("Colour"), s=w3643, f=w3636) -> (s? t:f=w3645:T2)
        n179 = Select(t=Box_Colour_FGV_Colours."Black" ("Colour"), s=w3646, f=w3645) -> (s? t:f=w3648:T2)
        n180 = Select(t=Box_Colour_FGV_Colours."Red" ("Colour"), s=w3650, f=w3648) -> (s? t:f=w3635:T2)
        n181 = Bundle By Name(cluster=w3655, "Red"=w3650, "Black"=w3646, "Blue"=w3643, "Yellow"=w3642, "Green"=w3639, "Unknown"=w3652, "Image processing done"=w3651, "Colour"=w3635) -> (w3654:T1)
      }
      frame "-----ARM ACTIONS-----" {
      }
      frame "CLOSE CLAW" {
        n182 = call "Arduino Interfacing VI.vi"("Data to Write"=I2C_MASTER_WRITE_NEW_Type_Def."Close Claw", "AE Mode"=Arduino_Interfacing."Write to Arduino") -> ()  [unwired: 2 in, 2 out]
      }
      frame "OPEN CLAW" {
        n183 = call "Arduino Interfacing VI.vi"("Data to Write"=I2C_MASTER_WRITE_NEW_Type_Def."Open Claw", "AE Mode"=Arduino_Interfacing."Write to Arduino") -> ()  [unwired: 2 in, 2 out]
      }
      frame "Z STEPPER CAM HEIGHT" {
        n184 = call "Arduino Interfacing VI.vi"("Data to Write"=I2C_MASTER_WRITE_NEW_Type_Def."zStepper 6k", "AE Mode"=Arduino_Interfacing."Write to Arduino") -> ()  [unwired: 2 in, 2 out]
      }
      frame "Z STEPPER GRAB HEIGHT" {
        # ">>State Logic  >>"
        # ">>> Time cluster >>>"
        # ">>> Yaw >>>"
        # ">>> Stepper position >>>"
        # ">>> Encoders >>>"
        # ">>> Object detection >>>"
        # ">>> Ultrasonic Sensors Detect >>>"
        n185 = call "Arduino Interfacing VI.vi"("Data to Write"=I2C_MASTER_WRITE_NEW_Type_Def."zStepper 100", "AE Mode"=Arduino_Interfacing."Write to Arduino") -> ()  [unwired: 2 in, 2 out]
      }
      frame "Z STEPPER BOX HEIGHT" {
        # ">>> IR Sensors >>>"
        # ">>> Time cluster >>>"
        # ">>> Yaw >>>"
        # ">>> Stepper position >>>"
        # ">>> Encoders >>>"
        # ">>> Object detection >>>"
        # ">>> Ultrasonic Sensors Detect >>>"
        n186 = call "Arduino Interfacing VI.vi"("Data to Write"=I2C_MASTER_WRITE_NEW_Type_Def."zStepper 5k", "AE Mode"=Arduino_Interfacing."Write to Arduino") -> ()  [unwired: 2 in, 2 out]
      }
      frame "Y STEPPER CONTROL" {
        # ">>State Logic  >>"
        # ">>> yStepper command>>>"
        # ">>> Time cluster >>>"
        # ">>> Yaw >>>"
        # ">>> Stepper position >>>"
        # ">>> Encoders >>>"
        # ">>> Object detection >>>"
        # ">>> Ultrasonic Sensors Detect >>>"
        n187 = Unbundle By Name(w3747) -> ("yStepper desired"=w3746:u8)
        n188 = call "Arduino Interfacing VI.vi"("y Stepper value"=w3746, "Data to Write"=I2C_MASTER_WRITE_NEW_Type_Def."yStepper control", "AE Mode"=Arduino_Interfacing."Write to Arduino") -> ()  [unwired: 1 in, 2 out]
      }
      frame "READ STEPPER VALUES" {
        # ">>State Logic  >>"
        # ">>> Time cluster >>>"
        # ">>> Yaw >>>"
        # ">>> Stepper position >>>"
        # ">>> Encoders >>>"
        # ">>> Object detection >>>"
        # ">>> Ultrasonic Sensors Detect >>>"
        n189 = call "Arduino Interfacing VI.vi"("AE Mode"=Arduino_Interfacing."Read From Arduino") -> ("Arduino Data"=w3765:T17)  [unwired: 3 in, 1 out]
        n190 = Unbundle By Name(w3765) -> ("y Stepper Position"=w3764:u8, "z Stepper Position"=w3763:u8)
        n191 = Bundle By Name(cluster=w3768, "y Stepper Position"=w3764, "z Stepper Position"=w3763) -> (w3767:T7)
      }
      frame " -----TIMING-----" {
        # ">>State Logic  >>"
        # ">>> Time cluster >>>"
        # ">>> Yaw >>>"
        # ">>> Stepper position >>>"
        # ">>> Encoders >>>"
        # ">>> Object detection >>>"
        # ">>> Ultrasonic Sensors Detect >>>"
      }
      frame "SET TIMER 1" {
        w3784 = 1.0 ("Time Setting")
        # ">>State Logic  >>"
        # ">>> Time cluster >>>"
        # ">>> Yaw >>>"
        # ">>> Stepper position >>>"
        # ">>> Encoders >>>"
        # ">>> Object detection >>>"
        # ">>> Ultrasonic Sensors Detect >>>"
        n192 = Wait (ms)(milliseconds to wait=u32 250) -> ()  [unwired: 1 out]
        n193 = call "Elasped Timer.vi"("Time Setting"=w3784, "Action"=Elapsed_timer_control."Initialize") -> ()  [unwired: 6 in, 4 out]
        n194 = Bundle By Name(cluster=w3793, "Time up flag"=FALSE, "SET TIME TO CHECK"=w3784) -> (w3791:T3)
      }
      frame "SET TIMER 2" {
        w3800 = 2.0 ("Time Setting")
        # ">>State Logic  >>"
        # ">>> Time cluster >>>"
        # ">>> Yaw >>>"
        # ">>> Stepper position >>>"
        # ">>> Encoders >>>"
        # ">>> Object detection >>>"
        # ">>> Ultrasonic Sensors Detect >>>"
        n195 = Wait (ms)(milliseconds to wait=u32 250) -> ()  [unwired: 1 out]
        n196 = call "Elasped Timer.vi"("Time Setting"=w3800, "Action"=Elapsed_timer_control."Initialize") -> ()  [unwired: 6 in, 4 out]
        n197 = Bundle By Name(cluster=w3809, "Time up flag"=FALSE, "SET TIME TO CHECK"=w3800) -> (w3807:T3)
      }
      frame "SET TIMER 3" {
        w3816 = 3.0 ("Time Setting")
        # ">>State Logic  >>"
        # ">>> Time cluster >>>"
        # ">>> Yaw >>>"
        # ">>> Stepper position >>>"
        # ">>> Encoders >>>"
        # ">>> Object detection >>>"
        # ">>> Ultrasonic Sensors Detect >>>"
        n198 = Wait (ms)(milliseconds to wait=u32 250) -> ()  [unwired: 1 out]
        n199 = call "Elasped Timer.vi"("Time Setting"=w3816, "Action"=Elapsed_timer_control."Initialize") -> ()  [unwired: 6 in, 4 out]
        n200 = Bundle By Name(cluster=w3825, "Time up flag"=FALSE, "SET TIME TO CHECK"=w3816) -> (w3823:T3)
      }
      frame "SET TIMER 4" {
        w3832 = 4.0 ("Time Setting")
        # ">>State Logic  >>"
        # ">>> Time cluster >>>"
        # ">>> Yaw >>>"
        # ">>> Stepper position >>>"
        # ">>> Encoders >>>"
        # ">>> Object detection >>>"
        # ">>> Ultrasonic Sensors Detect >>>"
        n201 = call "Elasped Timer.vi"("Time Setting"=w3832, "Action"=Elapsed_timer_control."Initialize") -> ()  [unwired: 6 in, 4 out]
        n202 = Wait (ms)(milliseconds to wait=u32 250) -> ()  [unwired: 1 out]
        n203 = Bundle By Name(cluster=w3841, "Time up flag"=FALSE, "SET TIME TO CHECK"=w3832) -> (w3839:T3)
      }
      frame "SET TIMER 5" {
        w3849 = 5.0 ("Time Setting")
        # ">>State Logic  >>"
        # ">>> Time cluster >>>"
        # ">>> Yaw >>>"
        # ">>> Stepper position >>>"
        # ">>> Encoders >>>"
        # ">>> Object detection >>>"
        # ">>> Ultrasonic Sensors Detect >>>"
        n204 = call "Elasped Timer.vi"("Time Setting"=w3849, "Action"=Elapsed_timer_control."Initialize") -> ("Time Out?!"=w3848:bool)  [unwired: 6 in, 3 out]
        n205 = Wait (ms)(milliseconds to wait=u32 250) -> ()  [unwired: 1 out]
        n206 = Bundle By Name(cluster=w3857, "Time up flag"=w3848, "SET TIME TO CHECK"=w3849) -> (w3856:T3)
      }
      frame "START TIMER" {
        # ">>State Logic  >>"
        # ">>> Time cluster >>>"
        # ">>> Yaw >>>"
        # ">>> Stepper position >>>"
        # ">>> Encoders >>>"
        # ">>> Object detection >>>"
        # ">>> Ultrasonic Sensors Detect >>>"
        n207 = call "Elasped Timer.vi"("Action"=Elapsed_timer_control."Start") -> ("Time Out?!"=w3868:bool)  [unwired: 7 in, 3 out]
        n208 = Bundle By Name(cluster=w3871, "Time up flag"=w3868) -> (w3870:T3)
      }
      frame "-----MISC-----" {
        # ">>> Box Colour Detection >>>"
        # ">>> Line Sensor Cluster>>>"
        # ">>> IR Sensors >>>"
        # ">>> Time cluster >>>"
        # ">>> Object detection >>>"
        # ">>> Yaw >>>"
        # ">>> Ultrasonic Sensors Detect >>>"
        # ">>> Encoders >>>"
        # ">>> Stepper position >>>"
      }
      frame "Task 9" {
        # ">>> Box Colour Detection >>>"
        # ">>> Line Sensor Cluster>>>"
        # ">>> IR Sensors >>>"
        # ">>> Time cluster >>>"
        # ">>> Object detection >>>"
        # ">>> Yaw >>>"
        # ">>> Ultrasonic Sensors Detect >>>"
        # ">>> Encoders >>>"
        # ">>> Stepper position >>>"
        n209 = call "Colour Processing Test Env.vi"() -> ("Colour scan time out?"=w3897:bool, "Colour output boolean cluster"=w3895:T47)  [unwired: 10 in]
        n210 = Unbundle By Name(w3895) -> ("Red"=w3889:bool, "Black"=w3890:bool, "Blue"=w3891:bool, "Yellow"=w3892:bool, "Green"=w3893:bool, "No recognizable coolour"=w3894:bool)
        n211 = Bundle By Name(cluster=w3899, "Red"=w3889, "Black"=w3890, "Blue"=w3891, "Yellow"=w3892, "Green"=w3893, "Unknown"=w3894, "Image processing done"=w3897) -> (w3898:T1)
      }
    }
    "State Logic" <- w268
    "Image Processing Error" <- w235
    n212 = local read "TASK ENABLE"() -> (w262:bool)
    n213 = Not(x=w262) -> (.not. x?=w261:bool)
    n214 = case shown="True" w269 {
      tunnel: w226 -> [w300 w354]
      tunnel: w276 -> [w296 w356]
      tunnel: [w300 w354] -> w281
      tunnel: [w296 w357] -> w280
      tunnel: w277 -> [_ w352]
      tunnel: w279 -> [_ w353]
      tunnel: w274 -> [w299 w359]
      tunnel: [w299 w359] -> w273
      tunnel: "STOP TASK" -> [_ w342]
      tunnel: w268 -> [w298 w358]
      tunnel: [w298 w355] -> w267
      tunnel: w264 -> [w297 w348]
      tunnel: [w297 w348] -> w263
      tunnel: w261 -> [_ w343]
      tunnel: [w295 w340] -> w260
      tunnel: w259 -> [w295 w339]
      tunnel: w257 -> [w294 w336]
      tunnel: [w294 w336] -> w256
      tunnel: w254 -> [w293 w332]
      tunnel: [w293 w332] -> w253
      tunnel: w251 -> [w292 w330]
      tunnel: [w292 w330] -> w250
      tunnel: w248 -> [w291 w328]
      tunnel: [w291 w328] -> w247
      tunnel: w246 -> [w290 w327]
      tunnel: [w290 w326] -> w245
      tunnel: [_ w324] -> w244
      tunnel: w242 -> [w289 w322]
      tunnel: [w289 w322] -> w241
      tunnel: w240 -> [w288 w321]
      tunnel: [w288 w320] -> w239
      tunnel: w237 -> [w287 w317]
      tunnel: [w287 w317] -> w236
      tunnel: [w286 w316] -> w234
      tunnel: w232 -> [w286 w315]
      tunnel: [_ w313] -> w231
      tunnel: [_ w312] -> w230
      tunnel: [_ w311] -> w229
      tunnel: w227 -> [w285 w310]
      tunnel: [w285 w310] -> w225
      tunnel: [_ w301] -> w224
      frame False {
        # ">>> Box Colour Detection >>>"
        # ">>> Line Sensor Cluster>>>"
        # ">> Item Selection Bias >>"
        # ">>State Logic Queue Reference >>"
        # ">>Action states Queue Reference >>"
        # ">>True Stop Next State >>"
        # ">>State Logic  >>"
        # ">>> IR Sensors >>>"
        # ">>> Line Sensor Cluster>>>"
        # ">>> Line Sensor Cluster>>>"
        # ">>> Motor control cluster >>>"
        # ">>> yStepper command>>>"
        # ">>> Motor control cluster >>>"
        # ">>> yStepper command>>>"
        # ">>> Motor control cluster >>>"
        # ">>> IR Sensors >>>"
        # ">>> IR Sensors >>>"
        # ">>> yStepper command>>>"
        # ">>> Time cluster >>>"
        # ">>> Yaw >>>"
        # ">>> Stepper position >>>"
        # ">>> Encoders >>>"
        # ">>> Object detection >>>"
        # ">>> Ultrasonic Sensors Detect >>>"
        # ">>> Time cluster >>>"
        # ">>> Yaw >>>"
        # ">>> Stepper position >>>"
        # ">>> Encoders >>>"
        # ">>> Object detection >>>"
        # ">>> Ultrasonic Sensors Detect >>>"
      }
      frame True {
        # ">>State Logic Queue Reference >>"
        # ">>> Box Colour Detection >>>"
        # ">> Item Selection Bias >>"
        # ">>> IR Sensors >>>"
        # ">>> Line Sensor Cluster>>>"
        # ">>> Line Sensor Cluster>>>"
        # ">>> Motor control cluster >>>"
        # ">>> yStepper command>>>"
        # ">>> IR Sensors >>>"
        # ">>> Motor control cluster >>>"
        # ">>State Logic Queue Reference >>"
        # ">>Timeout>>"
        # ">>> yStepper command>>>"
        # ">>> Time cluster >>>"
        # ">>> Object detection >>>"
        # ">>> Yaw >>>"
        # ">>> Ultrasonic Sensors Detect >>>"
        # ">>> Encoders >>>"
        # ">>> Stepper position >>>"
        # ">>State Logic  >>"
        # ">>True Stop Next State >>"
        # ">>Action Queue>>"
        # ">> Manual override >>"
        # ">>> Time cluster >>>"
        # ">>> Yaw >>>"
        # ">>> Stepper position >>>"
        # ">>> Encoders >>>"
        # ">>> Object detection >>>"
        # ">>> Ultrasonic Sensors Detect >>>"
        # ">>Action Queue>>"
        # ">>State Logic Queue Reference >>"
        n215 = Or(x=w342, y=w343) -> (x .or. y?=w341:bool)
        n216 = Unbundle By Name(w322) -> ("Left IR Sensor"=w323:dbl, "Arm IR Sensor"=w319:dbl, "Bottom IR Sensor"=w314:dbl)
        n217 = Unbundle By Name(w317) -> ("Line Detected?"=w318:bool)
        n218 = Unbundle By Name(w328) -> ("Time up flag"=w329:bool)
        n219 = Unbundle By Name(w330) -> ("Yaw"=w331:dbl, "Compass"=w325:dbl)
        n220 = Unbundle By Name(w332) -> ("y Stepper Position"=w334:u8, "z Stepper Position"=w333:u8)
        n221 = Unbundle By Name(w348) -> ("xDistance"=w345:dbl, "yDistance"=w346:dbl, "wDistance"=w347:dbl)
        n222 = Unbundle By Name(w336) -> ("Recognized Object"=w335:bool, "Object X coordinate"=w338:dbl, "Object Y coordinate"=w337:dbl)
        n223 = Unbundle By Name(w359) -> ("PING_A"=w351:u8, "PING_B"=w350:u8, "PING_C"=w349:u8, "PING_D"=w344:u8)
        n224 = Unbundle By Name(w310) -> ("Red"=w309:bool, "Black"=w308:bool, "Blue"=w307:bool, "Yellow"=w306:bool, "Green"=w305:bool, "Unknown"=w304:bool, "Image processing done"=w303:bool, "Colour"=w302:T2)
        n225 = case shown="28" w358 {
          tunnel: [w364 w376 w390 w401 w519 w536 w582 w619 w674 w716 w764 w808 w863 w911 w955 w1015 w1056 w1099 w1148 w1191 w1244 w1282 w1334 w1378 w1422 w1452 w1470 w1518 w1559 w1608 w1661 w1700 w1749 w1792 w1845 w1883 w1935 w1971 w2020 w2063 w2113 w2157 w2204 w2261 w2302 w2354 w2403 w2445 w2500 w2554 w2592 w2638 w2687 w2728 w2772 w2820 w2866 w2913 w2954] -> w357
          tunnel: w356 -> [w364 w379 w391 w404 w521 w537 w583 w628 w672 w720 w765 w814 w856 w914 w962 w1005 w1059 w1105 w1147 w1194 w1234 w1288 w1324 w1373 w1413 w1452 w1460 w1521 w1565 w1607 w1660 w1706 w1748 w1795 w1835 w1889 w1925 w1975 w2027 w2068 w2118 w2162 w2206 w2259 w2303 w2355 w2405 w2455 w2510 w2553 w2596 w2644 w2686 w2732 w2776 w2824 w2873 w2918 w2964]
          tunnel: [State_Type_Definitions,_for_0.26g_versions_and_later_2."Idle" ("Enum") State_Type_Definitions,_for_0.26g_versions_and_later_2."Idle" ("Enum") w386 w403 State_Type_Definitions,_for_0.26g_versions_and_later_2."Shutdown" ("Enum") w538 w584 w626 w675 w717 w763 w809 w862 w912 w957 w1014 w1057 w1106 w1149 w1193 w1243 w1289 w1333 w1379 w1414 State_Type_Definitions,_for_0.26g_versions_and_later_2."Idle" ("Enum") w1469 w1519 w1566 w1609 w1662 w1707 w1750 w1794 w1844 w1890 w1934 w1972 w2021 w2064 w2114 w2158 w2203 w2262 w2301 w2353 w2404 w2450 w2511 w2555 w2593 w2639 w2688 w2729 w2773 w2821 w2867 w2914 w2959] -> w355
          tunnel: w354 -> [_ _ w389 w407 _ w542 w589 w622 w671 w721 w772 w813 w860 w915 w961 w1012 w1054 w1104 w1145 w1195 w1241 w1287 w1331 w1376 w1421 _ w1467 w1516 w1564 w1605 w1658 w1705 w1746 w1796 w1842 w1888 w1932 w1979 w2026 w2071 w2121 w2165 w2214 w2258 w2304 w2348 w2406 w2454 w2509 w2552 w2600 w2643 w2685 w2736 w2777 w2827 w2872 w2921 w2963]
          tunnel: w353 -> [_ _ _ w406 _ w541 w588 w621 w670 w722 w771 w812 w859 w908 w960 w1011 w1053 w1103 w1144 w1196 w1240 w1286 w1330 w1375 w1419 _ w1466 w1515 w1563 w1604 w1657 w1704 w1745 w1797 w1841 w1887 w1931 w1974 w2025 w2070 w2120 w2164 w2212 w2257 w2305 w2349 w2407 w2453 w2508 w2551 w2599 w2642 w2684 w2735 w2778 w2823 w2871 w2920 w2962]
          tunnel: w352 -> [_ _ w388 w402 _ w540 w587 w620 w669 w723 w770 w811 w858 w907 w959 w1013 w1055 w1102 w1143 w1197 w1242 w1285 w1332 w1374 w1420 _ w1468 w1517 w1562 w1603 w1656 w1703 w1744 w1798 w1843 w1886 w1933 w1978 w2024 w2069 w2119 w2163 w2213 w2256 w2306 w2350 w2408 w2452 w2507 w2550 w2598 w2641 w2683 w2734 w2779 w2826 w2870 w2919 w2961]
          tunnel: w341 -> [_ _ _ _ _ w527 w581 w627 w668 w724 w767 w807 w861 w913 w963 w1006 w1060 w1100 w1146 w1198 w1235 w1283 w1325 w1377 w1417 _ w1461 w1522 w1560 w1606 w1659 w1701 w1747 w1799 w1836 w1884 w1926 w1977 w2019 w2067 w2117 w2161 w2208 w2255 w2307 w2351 w2409 w2451 w2506 w2549 w2597 w2640 w2682 w2733 w2780 w2825 w2865 w2917 w2960]
          tunnel: w351 -> [_ _ _ _ _ _ _ _ _ _ _ _ _ _ _ _ _ _ _ _ _ _ _ _ _ _ _ _ _ _ _ _ _ _ _ _ _ _ _ _ _ _ _ _ _ _ _ _ _ _ _ _ _ _ _ _ _ _ _]
          tunnel: w350 -> [_ _ _ _ _ _ _ _ w667 _ _ _ w852 w896 w953 _ _ _ _ _ _ _ _ _ _ _ _ w1508 _ _ _ _ _ _ _ _ _ _ _ _ _ _ _ _ _ _ _ _ w2504 _ _ _ _ _ _ _ _ _ _]
          tunnel: w349 -> [_ _ _ _ _ _ _ _ w666 _ _ _ w853 w897 w954 _ _ _ _ _ _ _ _ _ _ _ _ w1509 _ _ _ _ _ _ _ _ _ _ _ _ _ _ _ _ _ _ _ _ w2505 _ _ _ _ _ _ _ _ _ _]
          tunnel: w347 -> [_ _ _ _ _ _ _ _ _ _ w769 _ _ _ _ _ _ _ _ _ _ _ _ _ _ _ _ _ _ _ _ _ _ _ _ _ _ _ _ _ _ _ _ _ _ w2346 _ w2448 _ _ _ _ _ _ _ _ _ _ w2957]
          tunnel: w346 -> [_ _ _ _ _ w535 w580 _ _ w715 _ _ _ _ w958 _ _ _ _ _ _ _ _ _ _ _ _ _ _ _ _ _ _ _ _ _ _ _ _ _ _ _ _ _ _ _ _ _ w2496 _ _ _ _ _ _ _ _ _ _]
          tunnel: w345 -> [_ _ _ _ _ _ _ _ _ _ _ _ _ w902 _ _ _ _ _ _ _ _ _ _ _ _ _ _ _ _ w1647 _ _ _ _ _ _ _ _ _ _ _ _ w2248 _ _ _ _ _ _ _ _ w2681 _ _ _ _ _ _]
          tunnel: w344 -> [_ _ _ _ _ _ _ _ _ _ _ _ _ _ _ _ _ _ _ _ _ _ _ _ _ _ _ _ _ _ _ _ _ _ _ _ _ _ _ _ _ _ _ _ _ _ _ _ _ _ _ _ _ _ _ _ _ _ _]
          tunnel: [State_Type_Definitions,_for_0.26g_versions_and_later_2."Idle" ("Enum") State_Type_Definitions,_for_0.26g_versions_and_later_2."Idle" ("Enum") State_Type_Definitions,_for_0.26g_versions_and_later_2."Idle" ("Enum") State_Type_Definitions,_for_0.26g_versions_and_later_2."Idle" ("Enum") State_Type_Definitions,_for_0.26g_versions_and_later_2."Shutdown" ("Enum") w533 w578 w625 w673 w718 w760 w806 w855 w910 w956 w1016 w1058 w1098 w1150 w1192 w1245 w1281 w1335 w1380 w1415 w1454 w1471 w1520 w1558 w1610 w1663 w1699 w1751 w1793 w1846 w1882 w1936 w1973 w2022 w2066 w2116 w2160 w2202 w2260 w2300 w2352 w2402 w2449 w2512 w2556 w2594 w2637 w2689 w2730 w2774 w2822 w2868 w2916 w2958] -> w340
          tunnel: w339 -> [_ _ w386 _ _ _ _ _ _ _ _ _ _ _ _ _ _ _ _ _ _ _ _ _ _ w1454 _ _ _ _ _ _ _ _ _ _ _ _ _ _ _ _ _ _ _ _ _ _ _ _ _ _ _ _ _ _ _ _ _]
          tunnel: w335 -> [_ _ _ _ _ _ _ _ _ _ _ _ _ _ _ _ _ _ _ _ _ _ _ _ w1416 _ _ _ _ _ _ _ _ _ _ _ _ _ _ _ _ _ _ _ _ _ _ _ _ _ _ _ _ _ _ _ _ _ _]
          tunnel: w338 -> [_ _ _ _ _ _ _ _ _ _ _ _ _ _ _ _ _ _ _ _ _ _ _ _ _ _ _ _ _ _ w1653 _ _ _ _ _ _ _ _ _ _ _ _ _ _ _ _ _ _ _ _ _ _ _ _ _ _ _ _]
          tunnel: w337 -> [_ _ _ _ _ _ _ _ _ _ _ _ _ _ _ _ _ _ _ w1187 _ _ _ _ _ _ _ _ _ _ _ _ _ w1788 _ _ _ _ _ _ _ _ _ _ _ _ _ _ _ _ _ _ _ _ _ _ _ _ _]
          tunnel: w334 -> [_ _ _ _ _ _ _ _ _ _ _ _ _ _ _ _ _ _ _ w1186 _ _ _ _ _ _ _ _ _ _ _ _ _ w1787 _ _ _ _ _ _ _ _ _ _ _ _ _ _ _ _ _ _ _ _ _ _ _ _ _]
          tunnel: w333 -> [_ _ _ _ _ _ _ w624 _ _ _ w804 _ _ _ w1009 _ w1094 _ _ w1238 _ w1328 w1372 _ _ w1464 _ _ _ _ _ _ _ w1839 _ w1929 w1976 _ _ _ _ _ _ _ _ _ _ _ _ _ _ _ _ _ _ _ _ _]
          tunnel: w331 -> [_ _ _ _ _ _ _ _ _ _ _ _ _ _ _ _ _ _ _ _ _ _ _ _ _ _ _ _ _ _ _ _ _ _ _ _ _ _ _ _ _ _ _ _ _ _ _ _ _ _ _ _ _ _ _ _ _ _ _]
          tunnel: w329 -> [_ _ _ _ _ _ _ _ _ _ _ _ _ _ _ _ w1048 _ w1140 _ _ w1279 _ _ _ _ _ _ w1556 w1600 _ w1697 w1741 _ _ w1880 _ _ _ _ _ _ _ _ _ _ _ _ _ _ w2595 w2636 _ w2731 w2775 _ _ _ _]
          tunnel: w327 -> [w362 w374 w385 w399 w517 w532 w577 w623 w665 w719 w759 w805 w854 w906 w952 w1004 w1051 w1097 w1141 w1189 w1233 w1280 w1323 w1369 w1412 w1455 w1459 w1513 w1557 w1601 w1654 w1698 w1742 w1790 w1834 w1881 w1924 w1970 w2023 w2065 w2115 w2159 w2211 w2254 w2309 w2357 w2411 w2457 w2514 w2558 w2602 w2646 w2694 w2738 w2782 w2819 w2869 w2915 w2966]
          tunnel: [w362 w373 w385 w399 w517 w532 w577 w623 w665 w719 w759 w805 w854 w906 w952 w1004 w1051 w1097 w1141 w1188 w1233 w1280 w1323 w1369 w1412 w1455 w1459 w1513 w1557 w1601 w1654 w1698 w1742 w1789 w1834 w1881 w1924 w1970 w2023 w2065 w2115 w2159 w2211 w2254 w2309 w2357 w2411 w2457 w2514 w2558 w2602 w2646 w2694 w2738 w2782 w2819 w2869 w2915 w2966] -> w326
          tunnel: w325 -> [_ _ _ _ _ _ _ _ _ _ _ _ _ _ _ _ _ _ _ _ _ _ _ _ _ _ _ _ _ _ _ _ _ _ _ _ _ _ w2018 _ _ _ _ _ _ _ _ _ _ _ _ _ _ _ _ _ w2864 _ _]
          tunnel: [_ _ _ TRUE _ _ _ _ _ _ _ _ _ _ _ _ _ _ _ _ _ _ _ _ _ _ _ _ _ _ _ _ _ _ _ _ _ _ _ _ _ _ _ _ _ _ _ _ _ _ _ _ _ _ _ _ _ _ _] -> w324
          tunnel: w323 -> [_ _ _ _ _ _ _ _ _ _ _ _ _ _ _ _ _ _ _ _ _ _ _ _ _ _ _ _ _ _ _ _ _ _ _ _ _ _ _ _ _ _ _ _ _ _ _ _ _ _ _ _ _ _ _ _ _ _ _]
          tunnel: w321 -> [w361 w371 w384 w397 w516 w531 w576 w618 w664 w712 w758 w801 w847 w895 w951 w1003 w1050 w1096 w1139 w1183 w1232 w1278 w1322 w1368 w1411 w1456 w1458 w1507 w1555 w1599 w1650 w1696 w1740 w1784 w1833 w1879 w1923 w1969 w2014 w2062 w2112 w2156 w2210 w2253 w2311 w2359 w2413 w2459 w2516 w2560 w2604 w2648 w2696 w2740 w2784 w2818 w2860 w2912 w2968]
          tunnel: [w361 w370 w384 w397 w516 w531 w576 w618 w664 w712 w758 w801 w847 w895 w951 w1003 w1050 w1096 w1139 w1183 w1232 w1278 w1322 w1368 w1411 w1456 w1458 w1507 w1555 w1599 w1649 w1696 w1740 w1784 w1833 w1879 w1923 w1969 w2014 w2062 w2112 w2156 w2210 w2253 w2311 w2359 w2413 w2459 w2516 w2560 w2604 w2648 w2696 w2740 w2784 w2818 w2860 w2912 w2968] -> w320
          tunnel: w319 -> [_ _ _ _ _ _ _ _ _ _ _ _ _ _ _ _ _ _ _ _ _ _ _ _ _ _ _ _ _ _ _ _ _ _ _ _ _ _ _ _ w2110 _ _ _ _ _ w2398 _ w2502 _ _ _ _ _ _ _ _ _ _]
          tunnel: w318 -> [_ _ _ _ _ w528 _ _ _ _ _ _ _ _ w949 _ _ _ _ _ _ _ _ _ _ _ _ _ _ _ _ _ _ _ _ _ _ _ _ w2061 _ w2154 _ w2249 _ _ _ _ _ w2548 _ _ w2680 _ _ _ _ _ _]
          tunnel: [w360 w366 w383 w396 w515 w530 w575 w617 w663 w711 w757 w800 w846 w894 w950 w1002 w1049 w1095 w1138 w1182 w1231 w1277 w1321 w1367 w1410 w1451 w1457 w1506 w1554 w1598 w1642 w1695 w1739 w1783 w1832 w1878 w1922 w1968 w2013 w2060 w2109 w2155 w2209 w2252 w2310 w2358 w2412 w2458 w2515 w2559 w2603 w2647 w2695 w2739 w2783 w2817 w2859 w2911 w2967] -> w316
          tunnel: w315 -> [w360 w366 w383 _ w515 w530 w575 w617 w663 w711 w757 w800 w846 w894 w950 w1002 w1049 w1095 w1138 w1182 w1231 w1277 w1321 w1367 w1410 w1451 w1457 w1506 w1554 w1598 w1642 w1695 w1739 w1783 w1832 w1878 w1922 w1968 w2013 w2060 w2109 w2155 w2209 w2252 w2310 w2358 w2412 w2458 w2515 w2559 w2603 w2647 w2695 w2739 w2783 w2817 w2859 w2911 w2967]
          tunnel: w314 -> [_ _ _ _ _ _ _ _ _ _ _ _ _ _ _ _ _ _ _ _ _ _ _ _ _ _ _ w1505 _ _ _ _ _ _ _ _ _ _ _ _ w2108 _ _ _ _ _ w2395 _ _ _ _ _ _ _ _ _ _ w2908 _]
          tunnel: [_ _ _ _ _ _ _ _ w662 _ _ _ _ _ _ _ _ _ _ _ _ _ _ _ _ _ _ _ _ _ _ _ _ _ _ _ _ _ _ _ _ _ _ _ _ _ _ _ w2491 _ _ _ _ _ _ _ _ _ _] -> w313
          tunnel: [_ _ _ _ _ _ _ _ _ _ _ _ _ _ _ _ _ _ _ _ _ _ _ _ _ _ _ _ _ _ _ _ _ _ _ _ _ _ _ _ w2106 _ _ _ _ _ w2391 _ _ _ _ _ _ _ _ _ _ w2906 _] -> w312
          tunnel: [_ _ _ _ _ _ _ _ _ _ _ _ _ _ _ _ _ _ _ _ _ _ _ _ _ _ _ _ _ _ _ _ _ _ _ _ _ _ _ _ w2105 _ _ _ _ _ w2392 _ _ _ _ _ _ _ _ _ _ _ _] -> w311